vi "Graph Builder GUI - 6Dsupported.vi"() -> ()   [LabVIEW 2019]
uses:
  AxisMenu--Enum.ctl
  <vilib>/Utility/file.llb/Read Delimited Spreadsheet (string).vi
panel:
  out "Not Normalized":T1(array[cluster])
  out "Normalized":T1(array[cluster])
  out "Time Left (min)":dbl=54754.644
  out "Percent Complete":dbl(slide) scale=0.0..1.0
  in  "Axis Menu Type Def":T2 caption="Axis Menu" items=["<Ignore>", "<X Axis>", "<Y Axis>", "<Color Axis>", "<Time Axis>", "<Supra-X Scroll>", "<Supra-Y Scroll>"]
  in  "Normalize? (F)":bool
  in  "Path to Cleaned Data File":path=path "D:/Ian_s Dropbox/Dropbox/PostDoc/Programs/Data/2020-01-23 BigSlab2 Merged CLEAN  v01"
  in  "Axis Menus 2":T3={"Axis Menu 1"=1, "Axis Menu 2"=3, "Axis Menu 3"=0, "Axis Menu 4"=7, "Axis Menu 5"=9, "Axis Menu 6"=0, "Axis Menu 7"=0, "Axis Menu 8"=0, "Axis Menu 9"=4, "Axis Menu 10"=2, "Axis Menu 11"=0, "Axis Menu 12"=0} {"Axis Menu 12" items=["<Ignore>", "<X Axis>", "<Y Axis>", "<Color Axis>", "<Time Axis>", "<Supra-X Scroll>", "<Supra-Y Scroll>", "3000"]; "Axis Menu 11" items=["<Ignore>", "<X Axis>", "<Y Axis>", "<Color Axis>", "<Time Axis>", "<Supra-X Scroll>", "<Supra-Y Scroll>", "3.950000E+0", "4.300000E+0", "4.650000E+0", "5.000000E+0"]; "Axis Menu 10" items=["<Ignore>", "<X Axis>", "<Y Axis>", "<Color Axis>", "<Time Axis>", "<Supra-X Scroll>", "<Supra-Y Scroll>", "0.000000E+0"]; "Axis Menu 9" items=["<Ignore>", "<X Axis>", "<Y Axis>", "<Color Axis>", "<Time Axis>", "<Supra-X Scroll>", "<Supra-Y Scroll>", "0.000000E+0"]; "Axis Menu 8" items=["<Ignore>", "<X Axis>", "<Y Axis>", "<Color Axis>", "<Time Axis>", "<Supra-X Scroll>", "<Supra-Y Scroll>", "1.000000E-4"]; "Axis Menu 7" items=["<Ignore>", "<X Axis>", "<Y Axis>", "<Color Axis>", "<Time Axis>", "<Supra-X Scroll>", "<Supra-Y Scroll>", "1.000000E+0"]; "Axis Menu 6" items=["<Ignore>", "<X Axis>", "<Y Axis>", "<Color Axis>", "<Time Axis>", "<Supra-X Scroll>", "<Supra-Y Scroll>", "1.000000E+0", "2.000000E+0", "3.000000E+0"]; "Axis Menu 5" items=["<Ignore>", "<X Axis>", "<Y Axis>", "<Color Axis>", "<Time Axis>", "<Supra-X Scroll>", "<Supra-Y Scroll>", "9.200000E-1"]; "Axis Menu 4" items=["<Ignore>", "<X Axis>", "<Y Axis>", "<Color Axis>", "<Time Axis>", "<Supra-X Scroll>", "<Supra-Y Scroll>", "1.000000E-9", "3.500000E-1", "7.000000E-1", "1.050000E+0"]; "Axis Menu 3" items=["<Ignore>", "<X Axis>", "<Y Axis>", "<Color Axis>", "<Time Axis>", "<Supra-X Scroll>", "<Supra-Y Scroll>", "5.000000E+0"]; "Axis Menu 2" items=["<Ignore>", "<X Axis>", "<Y Axis>", "<Color Axis>", "<Time Axis>", "<Supra-X Scroll>", "<Supra-Y Scroll>", "SLAB"]; "Axis Menu 1" items=["<Ignore>", "<X Axis>", "<Y Axis>", "<Color Axis>", "<Time Axis>", "<Supra-X Scroll>", "<Supra-Y Scroll>", "2.0"]}
  in  "Color 1":u32(colorbox)
  in  "Color 2":u32(colorbox)=16711680
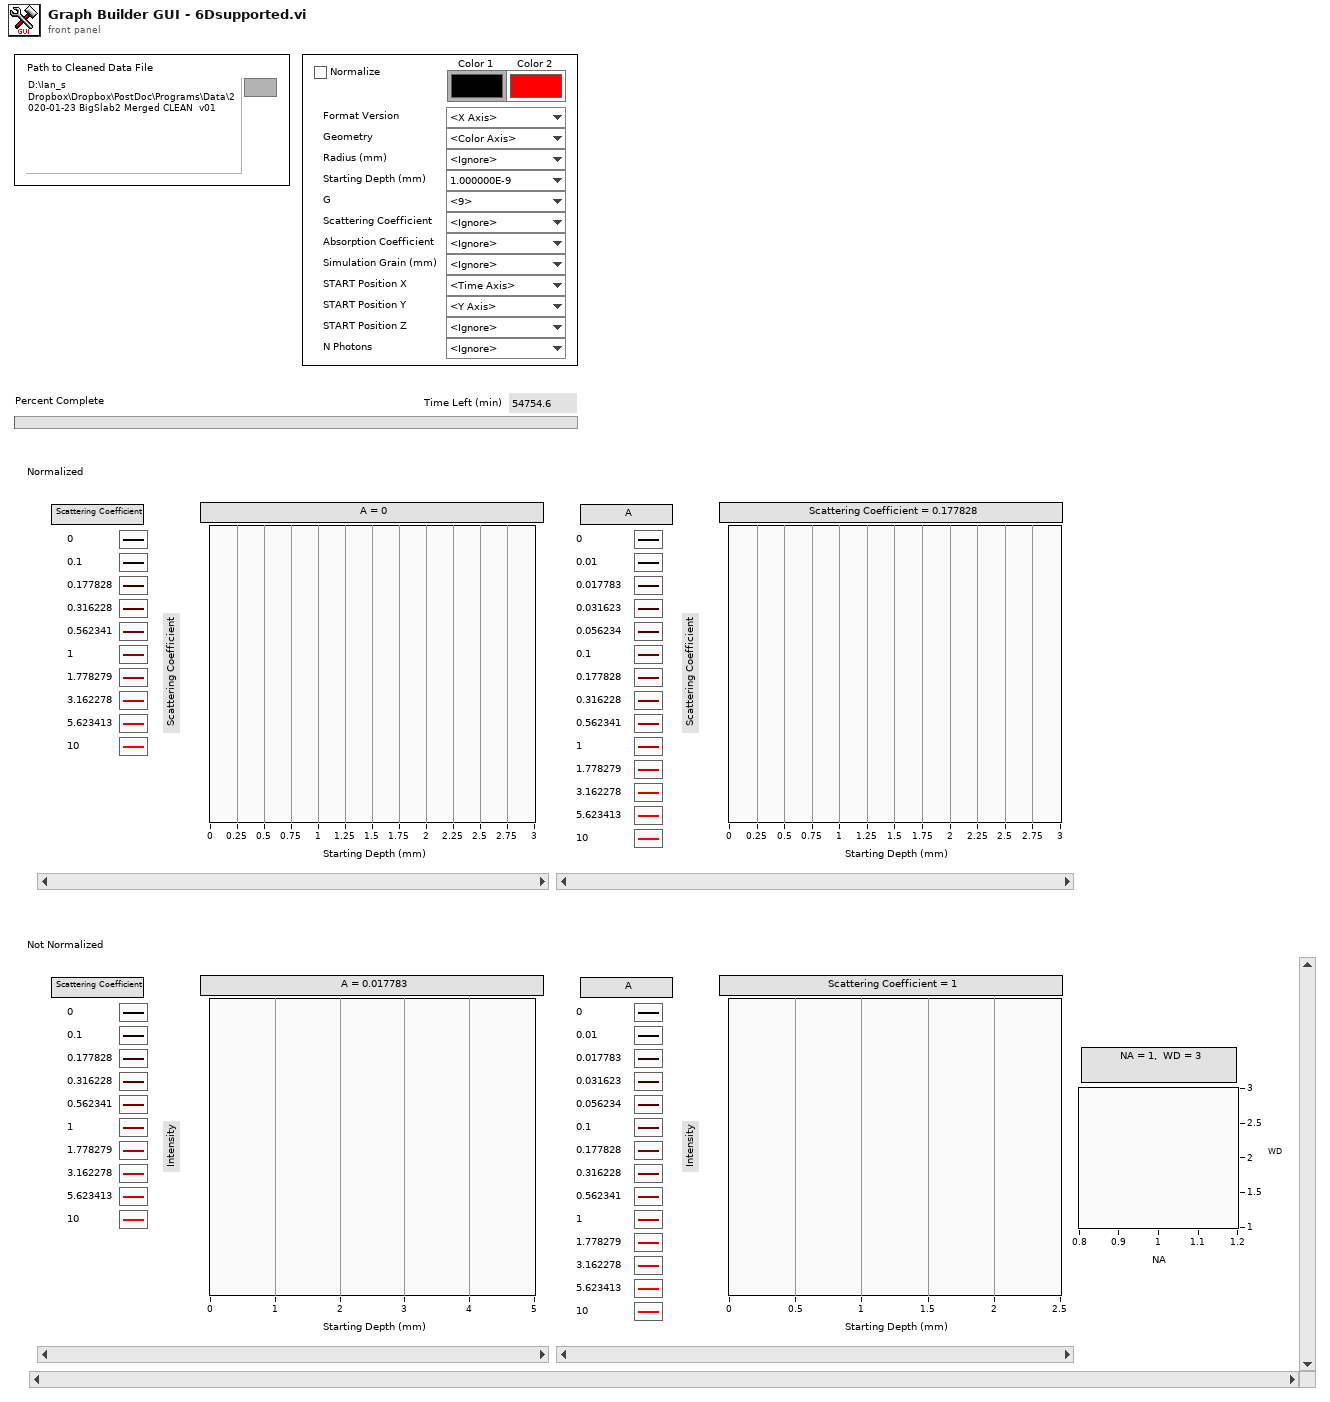
[diagram p1: front panel]
types:
  T1 = cluster{"Slab C=A, T=S 2":cluster{"Color and Time Graph":cluster{dbl[], dbl[]}[], "String":string, "String 2":string}[], "Slab C=S, T=A":cluster{"Color and Time Flipped Graph":cluster{dbl[], dbl[]}[], "String":string, "String 2":string}[], "Supra-Space Label":string, "Supra-Space Mini Map":cluster{dbl[], dbl[]}[]}[][]
  T2 = typedef "AxisMenu--Enum.ctl" = u16
  T3 = cluster{"Axis Menu 1":u16, "Axis Menu 2":u16, "Axis Menu 3":u16, "Axis Menu 4":u16, "Axis Menu 5":u16, "Axis Menu 6":u16, "Axis Menu 7":u16, "Axis Menu 8":u16, "Axis Menu 9":u16, "Axis Menu 10":u16, "Axis Menu 11":u16, "Axis Menu 12":u16}
  T4 = cluster{cluster{dbl[], dbl[]}[], string, "Caption.Text":string}[]
  T5 = cluster{"Graph":cluster{cluster{dbl[], dbl[]}[], string, "Caption.Text":string}[], "Graph":cluster{cluster{dbl[], dbl[]}[], string, "Caption.Text":string}[], string, cluster{dbl[], dbl[]}[]}
  T6 = cluster{"Graph":cluster{cluster{dbl[], dbl[]}[], string, "Caption.Text":string}[], "Graph":cluster{cluster{dbl[], dbl[]}[], string, "Caption.Text":string}[], string, cluster{dbl[], dbl[]}[]}[][]
  T7 = cluster{"Graph":cluster{cluster{dbl[], dbl[]}[], string, "Caption.Text":string}[], "Graph":cluster{cluster{dbl[], dbl[]}[], string, "Caption.Text":string}[], string, "XY Graph in Array":cluster{i32[], i32[]}[]}
  T8 = cluster{"Graph":cluster{cluster{dbl[], dbl[]}[], string, "Caption.Text":string}[], "Graph":cluster{cluster{dbl[], dbl[]}[], string, "Caption.Text":string}[], string, "XY Graph in Array":cluster{i32[], i32[]}[]}[]
  T9 = cluster{"Graph":cluster{cluster{dbl[], dbl[]}[], string, "Caption.Text":string}[], "Graph":cluster{cluster{dbl[], dbl[]}[], string, "Caption.Text":string}[], string, "XY Graph in Array":cluster{i32[], i32[]}[]}[][]
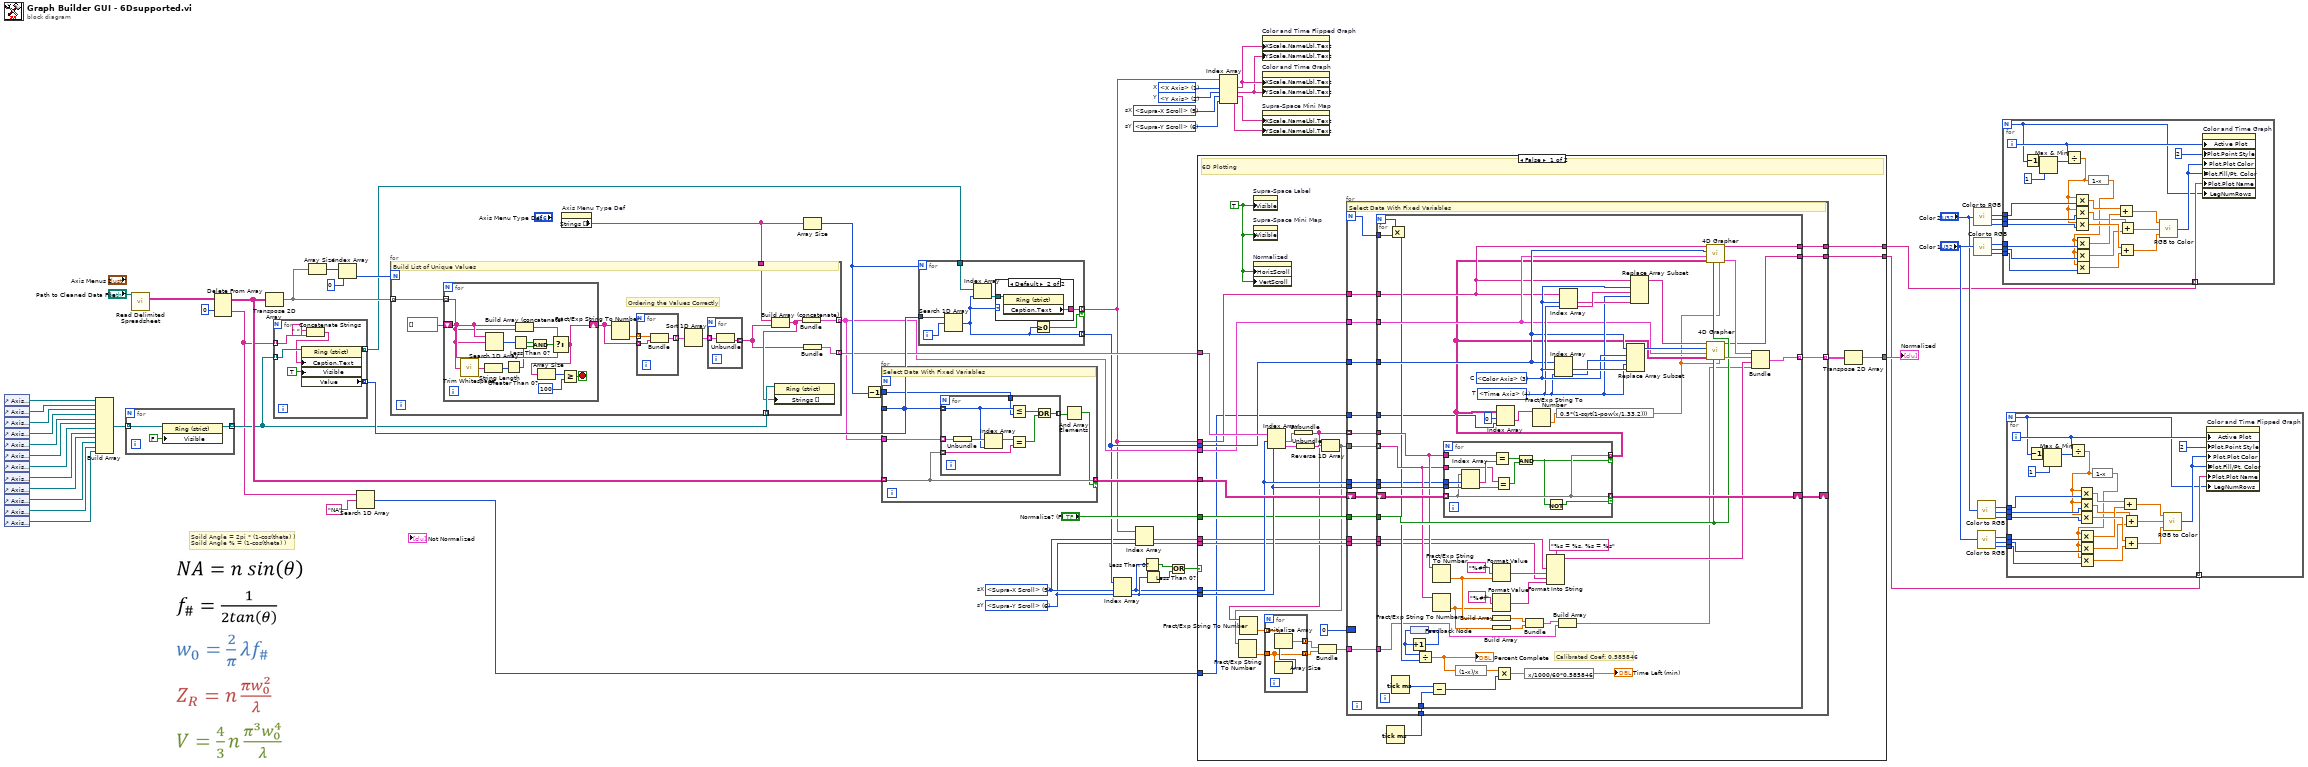
[diagram p0: block diagram]
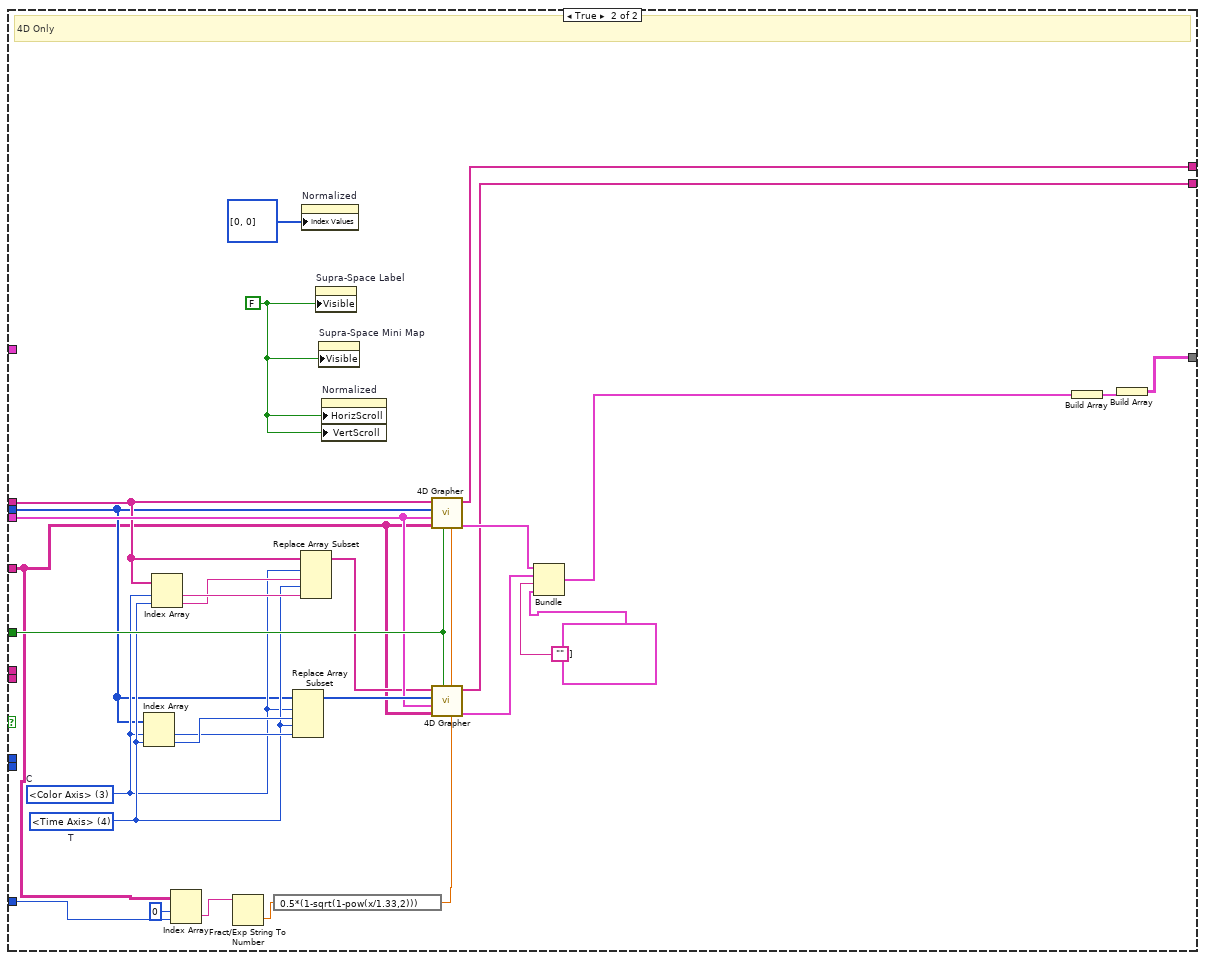
[diagram p2: hidden frame]
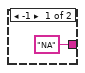
[diagram p3: hidden frame]
diagram:
  w6 = T2 1 items=["<Ignore>", "<X Axis>", "<Y Axis>", "<Color Axis>", "<Time Axis>", "<Supra-X Scroll>", "<Supra-Y Scroll>"]  # X
  w9 = T2 6 items=["<Ignore>", "<X Axis>", "<Y Axis>", "<Color Axis>", "<Time Axis>", "<Supra-X Scroll>", "<Supra-Y Scroll>"]  # sY
  w10 = T2 5 items=["<Ignore>", "<X Axis>", "<Y Axis>", "<Color Axis>", "<Time Axis>", "<Supra-X Scroll>", "<Supra-Y Scroll>"]  # sX
  w13 = T2 6 items=["<Ignore>", "<X Axis>", "<Y Axis>", "<Color Axis>", "<Time Axis>", "<Supra-X Scroll>", "<Supra-Y Scroll>"]  # sY
  w14 = T2 5 items=["<Ignore>", "<X Axis>", "<Y Axis>", "<Color Axis>", "<Time Axis>", "<Supra-X Scroll>", "<Supra-Y Scroll>"]  # sX
  w46 = T2 2 items=["<Ignore>", "<X Axis>", "<Y Axis>", "<Color Axis>", "<Time Axis>", "<Supra-X Scroll>", "<Supra-Y Scroll>"]  # Y
  # "Soild Angle = 2pi * (1-cos(theta) )\nSoild Angle % = (1-cos(theta) )"
  n1 = control-ref of="Axis Menu 1"() -> (w51:refnum<vi>)
  n2 = control-ref of="Axis Menu 2"() -> (w66:refnum<vi>)
  n3 = control-ref of="Axis Menu 3"() -> (w65:refnum<vi>)
  n4 = control-ref of="Axis Menu 4"() -> (w64:refnum<vi>)
  n5 = control-ref of="Axis Menu 5"() -> (w63:refnum<vi>)
  n6 = control-ref of="Axis Menu 6"() -> (w62:refnum<vi>)
  n7 = control-ref of="Axis Menu 7"() -> (w61:refnum<vi>)
  n8 = control-ref of="Axis Menu 8"() -> (w60:refnum<vi>)
  n9 = control-ref of="Axis Menu 9"() -> (w59:refnum<vi>)
  n10 = control-ref of="Axis Menu 10"() -> (w58:refnum<vi>)
  n11 = control-ref of="Axis Menu 11"() -> (w57:refnum<vi>)
  n12 = control-ref of="Axis Menu 12"() -> (w56:refnum<vi>)
  n13 = Build Array(w51, w66, w65, w64, w63, w62, w61, w60, w59, w58, w57, w56) -> (w55:refnum<vi>[])
  n14 = for {
    tunnel: w55 -> [w73] mode=indexing
    tunnel: [w71] -> w44 mode=indexing
    n15 = property on="Property Node" class="Ring (strict)"(reference=w73, "Visible"=FALSE) -> (reference out=w71:refnum<vi>)  [unwired: 1 in, 1 out]
  }
  n16 = call-poly <vilib>:"Read Delimited Spreadsheet.vi"("file path (dialog if empty)"="Path to Cleaned Data File") -> ("all rows"=w52:string[][])  [unwired: 9 in, 5 out]
  n17 = Delete From Array(array=w52, index (row)=0) -> (deleted portion=w3:string[], array with subset deleted=w50:string[][])  [unwired: 2 in]
  n18 = Transpose 2D Array(2D array=w50) -> (transposed array=w68:string[][])
  n19 = for {
    tunnel: w3 -> [w76] mode=indexing
    tunnel: w44 -> [w80] mode=indexing
    tunnel: [w78] -> w47 mode=indexing
    tunnel: [w77] -> w45 mode=indexing
    n20 = Concatenate Strings(" " ("string"), w76) -> (w74:string)
    n21 = property on="Property Node" class="Ring (strict)"(reference=w80, "Caption.Text"=w74, "Visible"=TRUE) -> (reference out=w77:refnum<vi>, "Value"=w78:u16)  [unwired: 1 in, 1 out]
  }
  n22 = Array Size(array=w68) -> (size(s)=w69:i32[])
  n23 = Index Array(array=w69, index=0) -> (element=w54:i32)
  n24 = Search 1D Array(1D array=w3, element="NA") -> (index of element=w1:i32)  [unwired: 1 in]
  n25 = property on="Axis Menu Type Def" class="Ring (strict)"() -> ("Strings []"=w49:string[])  [unwired: 2 in, 2 out]
  n26 = for {
    N: w54 -> [_]
    tunnel: w68 -> [w92] mode=indexing
    tunnel: [w90] -> w34 mode=indexing
    tunnel: w49 -> [w89]
    tunnel: w44 -> [w88] mode=indexing
    tunnel: [w86] -> w37 mode=indexing
    # "Ordering the Values Correctly"
    # "Build List of Unique Values"
    n27 = for {
      tunnel: w92 -> [w99] mode=indexing
      shift-right: [w106] -> w82
      shift-left: string[] [] -> [w110]
      stop <- w103 stop-if-true
      n28 = call <vilib>:"Trim Whitespace.vi"("string"=w99) -> ("trimmed string"=w98:string)  [unwired: 1 in]
      n29 = String Length(string=w98) -> (length=w102:i32)
      n30 = Search 1D Array(1D array=w110, element=w99) -> (index of element=w108:i32)  [unwired: 1 in]
      n31 = Greater Than 0?(x=w102) -> (x > 0?=w100:bool)
      n32 = Less Than 0?(x=w108) -> (x < 0?=w107:bool)
      n33 = Build Array (concatenate)(w110, w99) -> (w109:string[])
      n34 = And(x=w107, y=w100) -> (x .and. y?=w101:bool)
      n35 = Select(t=w109, s=w101, f=w110) -> (s? t:f=w106:string[])
      n36 = Array Size(array=w106) -> (size(s)=w105:i32)
      n37 = Greater Or Equal?(x=w105, y=100) -> (x >= y?=w103:bool)
    }
    n38 = Fract/Exp String To Number(string=w82) -> (number=w85:dbl[])  [unwired: 3 in, 1 out]
    n39 = for {
      tunnel: w85 -> [w97] mode=indexing
      tunnel: w82 -> [w96] mode=indexing
      tunnel: [w95] -> w84 mode=indexing
      n40 = Bundle(w97, w96) -> (w95:cluster{dbl, string})  [unwired: 1 in]
    }
    n41 = Sort 1D Array(array=w84) -> (sorted array=w83:cluster{dbl, string}[])
    n42 = for {
      tunnel: w83 -> [w94] mode=indexing
      tunnel: [w93] -> w81 mode=indexing
      n43 = Unbundle(w94) -> (w93:string)  [unwired: 1 out]
    }
    n44 = Build Array (concatenate)(w89, w81) -> (w87:string[])
    n45 = property on="Property Node" class="Ring (strict)"(reference=w88, "Strings []"=w87) -> ()  [unwired: 1 in, 2 out]
    n46 = Bundle(w87) -> (w90:cluster{string[]})  [unwired: 1 in]
    n47 = Bundle(w81) -> (w86:cluster{string[]})  [unwired: 1 in]
  }
  n48 = Array Size(array=w49) -> (size(s)=w43:i32)
  n49 = Decrement(x=w43) -> (x-1=w48:i32)
  n50 = for {
    tunnel: w50 -> [w115] mode=indexing
    tunnel: [w115] -> w35 mode=indexing if=w112
    tunnel: w47 -> [w116]
    tunnel: w34 -> [w114]
    tunnel: w48 -> [w111]
    # "Select Data With Fixed Variables"
    n51 = for {
      tunnel: w116 -> [w121] mode=indexing
      tunnel: w115 -> [w123] mode=indexing
      tunnel: w114 -> [w125] mode=indexing
      tunnel: [w118] -> w113 mode=indexing
      tunnel: w111 -> [w117]
      n52 = Unbundle(w125) -> (w124:string[])
      n53 = Index Array(array=w124, index=w121) -> (element=w122:string)
      n54 = Less Or Equal?(x=w121, y=w117) -> (x <= y?=w120:bool)
      n55 = Equal?(x=w122, y=w123) -> (x = y?=w119:bool)
      n56 = Or(x=w120, y=w119) -> (x .or. y?=w118:bool)
    }
    n57 = And Array Elements(Boolean array=w113) -> (logical AND=w112:bool)
  }
  n58 = for {
    N: w43 -> [_]
    tunnel: w47 -> [w132]
    tunnel: [w127] -> w33 mode=indexing
    tunnel: w45 -> [w129]
    tunnel: [w128] -> w15 mode=indexing if=w126
    i -> [w131]
    n59 = Search 1D Array(1D array=w132, element=w131) -> (index of element=w127:i32)  [unwired: 1 in]
    n60 = Index Array(array=w129, index=w127) -> (element=w130:refnum<vi>)
    n61 = case shown="Default" w127 {
      tunnel: w130 -> [_ w135]
      tunnel: ["NA" ("Caption.Text") w134] -> w128
      frame -1 {
      }
      frame Default {
        n62 = property on="Property Node" class="Ring (strict)"(reference=w135) -> ("Caption.Text"=w134:string)  [unwired: 1 in, 2 out]
      }
    }
    n63 = Greater Or Equal To 0?(x=w127) -> (x >= 0?=w126:bool)
  }
  n64 = Index Array(array=w33, index #1=w14, index #2=w13) -> (element #1=w38:i32, element #2=w39:i32)
  n65 = Index Array(array=w15, index #1=w14, index #2=w13) -> (element #1=w12:string, element #2=w11:string)
  n66 = Less Than 0?(x=w38) -> (x < 0?=w41:bool)
  n67 = Less Than 0?(x=w39) -> (x < 0?=w42:bool)
  n68 = Or(x=w41, y=w42) -> (x .or. y?=w40:bool)
  n69 = case shown="False" w40 {
    tunnel: "Normalize? (F)" -> [w154 w279]
    tunnel: w34 -> [w156 w278]
    tunnel: w35 -> [w163 w259]
    tunnel: w15 -> [w155 w273]
    tunnel: w33 -> [w157 w271]
    tunnel: w39 -> [w158 _]
    tunnel: w38 -> [w162 _]
    tunnel: w37 -> [w160 _]
    tunnel: [w142 w269] -> w32
    tunnel: [w151 w264] -> w17
    tunnel: [w150 w263] -> w16
    tunnel: w12 -> [w141 _]
    tunnel: w11 -> [w140 _]
    tunnel: w1 -> [w136 w258]
    frame False {
      w137 = TRUE ("Visible")
      # "6D Plotting"
      n70 = property on="Supra-Space Label" class="Str"("Visible"=w137) -> ()  [unwired: 2 in, 2 out]
      n71 = property on="Supra-Space Mini Map" class="XYGraph (strict)"("Visible"=w137) -> ()  [unwired: 2 in, 2 out]
      n72 = property on="Normalized" class="Arr (strict)"("HorizScroll"=w137, "VertScroll"=w137) -> ()  [unwired: 2 in, 2 out]
      n73 = Index Array(array=w160, index #1=w162, index #2=w158) -> (element #1=w161:cluster{string[]}, element #2=w159:cluster{string[]})
      n74 = Unbundle(w161) -> (w139:string[])
      n75 = Fract/Exp String To Number(string=w139) -> (number=w148:dbl[])  [unwired: 3 in, 1 out]
      n76 = Unbundle(w159) -> (w149:string[])
      n77 = Reverse 1D Array(array=w149) -> (reversed array=w138:string[])
      n78 = Fract/Exp String To Number(string=w138) -> (number=w147:dbl[])  [unwired: 3 in, 1 out]
      n79 = for {
        tunnel: w148 -> [w167] mode=indexing
        tunnel: w147 -> [w164]
        tunnel: [w166] -> w145 mode=concatenating
        tunnel: [w164] -> w144 mode=concatenating
        n80 = Array Size(array=w164) -> (size(s)=w165:i32)
        n81 = Initialize Array(w167, w165) -> (w166:dbl[])
      }
      n82 = Bundle(w145, w144) -> (w143:cluster{dbl[], dbl[]})  [unwired: 1 in]
      n83 = Tick Count (ms)() -> (millisecond timer value=w153:u32)
      n84 = for {
        N -> [w172]
        tunnel: w162 -> [w185]
        tunnel: w138 -> [w183]
        tunnel: w139 -> [w184] mode=indexing
        shift-right: [w181] -> _
        shift-left: w163 -> [w186]
        tunnel: w158 -> [w182]
        tunnel: w156 -> [w180]
        tunnel: w155 -> [w179]
        tunnel: w157 -> [w178]
        tunnel: w154 -> [w177]
        tunnel: w153 -> [w176]
        tunnel: [w175] -> w152 mode=indexing
        tunnel: [w174] -> w151
        tunnel: [w173] -> w150
        border: 0 -> [_]
        tunnel: w143 -> [w171]
        tunnel: w141 -> [w170]
        tunnel: w140 -> [w169]
        tunnel: w136 -> [w168]
        # "Select Data With Fixed Variables"
        n85 = for {
          N -> [w226]
          tunnel: w185 -> [w195]
          tunnel: w184 -> [w215]
          tunnel: w183 -> [w213] mode=indexing
          shift-right: [w240] -> w181
          shift-left: w186 -> [w242]
          tunnel: w182 -> [w241]
          tunnel: w180 -> [w227]
          tunnel: w179 -> [w196]
          tunnel: w178 -> [w229]
          tunnel: w177 -> [w228]
          tunnel: w176 -> [w224]
          tunnel: [w211] -> w175 mode=indexing
          tunnel: [w209] -> w174
          tunnel: [w208] -> w173
          tunnel: w172 -> [w206]
          tunnel: w171 -> [w199]
          tunnel: w170 -> [w194]
          tunnel: w169 -> [w193]
          tunnel: w168 -> [w188]
          w230 = T2 4 items=["<Ignore>", "<X Axis>", "<Y Axis>", "<Color Axis>", "<Time Axis>", "<Supra-X Scroll>", "<Supra-Y Scroll>"]  # T
          w231 = T2 3 items=["<Ignore>", "<X Axis>", "<Y Axis>", "<Color Axis>", "<Time Axis>", "<Supra-X Scroll>", "<Supra-Y Scroll>"]  # C
          # "Calibrated Coef: 0.585846"
          n86 = Multiply(x=w226, y=w206) -> (x*y=w207:i32)
          n87 = Tick Count (ms)() -> (millisecond timer value=w225:u32)
          n88 = feedback #1() -> (w204:i32)
          n89 = Increment(x=w204) -> (x+1=w205:i32)
          n90 = feedback-in #1(w205) -> ()
          n91 = Divide(x=w204, y=w207) -> (x/y=w223:dbl)
          "Percent Complete" <- w223
          n92 = Subtract(x=w225, y=w224) -> (x-y=w221:u32)
          n93 = Fract/Exp String To Number(string=w215) -> (number=w203:dbl)  [unwired: 3 in, 1 out]
          n94 = Fract/Exp String To Number(string=w213) -> (number=w202:dbl)  [unwired: 3 in, 1 out]
          n95 = for {
            tunnel: w242 -> [w245] mode=indexing
            tunnel: w215 -> [w253]
            tunnel: w213 -> [w248]
            tunnel: w241 -> [w252]
            tunnel: w195 -> [w251]
            tunnel: [w245] -> w240 mode=indexing if=w243
            tunnel: [w245] -> w189 mode=indexing if=w244
            n96 = Index Array(array=w245, index #1=w251, index #2=w252) -> (element #1=w249:string, element #2=w250:string)
            n97 = Equal?(x=w253, y=w249) -> (x = y?=w246:bool)
            n98 = Equal?(x=w248, y=w250) -> (x = y?=w247:bool)
            n99 = And(x=w246, y=w247) -> (x .and. y?=w244:bool)
            n100 = Not(x=w244) -> (.not. x?=w243:bool)
          }
          n101 = expression code="(1-x)/x"(w223) -> (w222:dbl)
          n102 = Format Value(format string="%#f", value (0)=w203) -> (output string=w218:string)  [unwired: 1 in]
          n103 = Build Array(w203) -> (w201:dbl[])
          n104 = Build Array(w202) -> (w200:dbl[])
          n105 = Format Value(format string="%#f", value (0)=w202) -> (output string=w212:string)  [unwired: 1 in]
          n106 = Multiply(x=w222, y=w221) -> (x*y=w220:dbl)
          n107 = Index Array(array=w189, index (row)=0 ("disabled index (row)"), index (col)=w188) -> (element=w191:string)
          n108 = expression code="x/1000/60*0.585846"(w220) -> (→"Time Left (min)":dbl)
          n109 = Bundle(w201, w200) -> (w198:cluster{dbl[], dbl[]})  [unwired: 1 in]
          n110 = Fract/Exp String To Number(string=w191) -> (number=w190:dbl)  [unwired: 3 in, 1 out]
          n111 = Format Into String(format string="%s = %s, %s = %s", w194, w218, w193, w212) -> (resulting string=w210:string)  [unwired: 2 in, 1 out]
          n112 = Index Array(array=w229, index #1=w231, index #2=w230) -> (element #1=w233:i32, element #2=w232:i32)
          n113 = expression code="0.5*(1-sqrt(1-pow(x/1.33,2)))"(w190) -> (w187:dbl)
          n114 = Build Array(w198, w199) -> (w197:cluster{dbl[], dbl[]}[])
          n115 = Index Array(array=w196, index #1=w231, index #2=w230) -> (element #1=w234:string, element #2=w235:string)
          n116 = Replace Array Subset(array=w229, new element #1=w232, index #1=w231, new element #2=w233, index #2=w230) -> (w237:i32[])
          n117 = Replace Array Subset(array=w196, new element #1=w235, index #1=w231, new element #2=w234, index #2=w230) -> (w236:string[])
          n118 = call "4D Grapher.vi"("Norm Factor (NaN: use first element)"=w187, "Normalize? (F)"=w228, "Pruned Data"=w189, "String Items from Axes Menus"=w227, "Axes Indexes"=w229, "Axes Names"=w196) -> ("Graph"=w239:T4, "Color Axis Titles"=w209:string[])  [unwired: 4 in]
          n119 = call "4D Grapher.vi"("Norm Factor (NaN: use first element)"=w187, "Normalize? (F)"=w228, "Pruned Data"=w189, "String Items from Axes Menus"=w227, "Axes Indexes"=w237, "Axes Names"=w236) -> ("Graph"=w238:T4, "Color Axis Titles"=w208:string[])  [unwired: 4 in]
          n120 = Bundle("Graph"=w239, "Graph"=w238, w210, w197) -> (w211:T5)  [unwired: 1 in]
        }
      }
      n121 = Transpose 2D Array(2D array=w152) -> (transposed array=w142:T6)
    }
    frame True {
      w260 = FALSE ("Visible")
      w275 = T2 4 items=["<Ignore>", "<X Axis>", "<Y Axis>", "<Color Axis>", "<Time Axis>", "<Supra-X Scroll>", "<Supra-Y Scroll>"]  # T
      w274 = T2 3 items=["<Ignore>", "<X Axis>", "<Y Axis>", "<Color Axis>", "<Time Axis>", "<Supra-X Scroll>", "<Supra-Y Scroll>"]  # C
      # "4D Only"
      n122 = Index Array(array=w271, index #1=w274, index #2=w275) -> (element #1=w281:i32, element #2=w282:i32)
      n123 = Index Array(array=w273, index #1=w274, index #2=w275) -> (element #1=w277:string, element #2=w276:string)
      n124 = Index Array(array=w259, index (row)=0 ("disabled index (row)"), index (col)=w258) -> (element=w256:string)
      n125 = Fract/Exp String To Number(string=w256) -> (number=w255:dbl)  [unwired: 3 in, 1 out]
      n126 = expression code="0.5*(1-sqrt(1-pow(x/1.33,2)))"(w255) -> (w254:dbl)
      n127 = Replace Array Subset(array=w271, new element #1=w282, index #1=w274, new element #2=w281, index #2=w275) -> (w280:i32[])
      n128 = Replace Array Subset(array=w273, new element #1=w276, index #1=w274, new element #2=w277, index #2=w275) -> (w272:string[])
      n129 = property on="Normalized" class="Arr (strict)"("Index Values"=u32[] [0, 0]) -> ()  [unwired: 2 in, 2 out]
      n130 = property on="Supra-Space Label" class="Str"("Visible"=w260) -> ()  [unwired: 2 in, 2 out]
      n131 = property on="Supra-Space Mini Map" class="XYGraph (strict)"("Visible"=w260) -> ()  [unwired: 2 in, 2 out]
      n132 = property on="Normalized" class="Arr (strict)"("HorizScroll"=w260, "VertScroll"=w260) -> ()  [unwired: 2 in, 2 out]
      n133 = call "4D Grapher.vi"("Norm Factor (NaN: use first element)"=w254, "Normalize? (F)"=w279, "Pruned Data"=w259, "String Items from Axes Menus"=w278, "Axes Indexes"=w271, "Axes Names"=w273) -> ("Graph"=w268:T4, "Color Axis Titles"=w264:string[])  [unwired: 4 in]
      n134 = call "4D Grapher.vi"("Norm Factor (NaN: use first element)"=w254, "Normalize? (F)"=w279, "Pruned Data"=w259, "String Items from Axes Menus"=w278, "Axes Indexes"=w280, "Axes Names"=w272) -> ("Graph"=w267:T4, "Color Axis Titles"=w263:string[])  [unwired: 4 in]
      n135 = Bundle("Graph"=w268, "Graph"=w267, "", "XY Graph in Array"=cluster{i32[], i32[]}[] []) -> (w265:T7)  [unwired: 1 in]
      n136 = Build Array(w265) -> (w270:T8)
      n137 = Build Array(w270) -> (w269:T9)
    }
  }
  "Normalized" <- w32
  n138 = Index Array(array=w15, index #1=w6, index #2=w46, index #3=w10, index #4=w9) -> (element #1=w5:string, element #2=w4:string, element #3=w8:string, element #4=w7:string)
  n139 = property on="Color and Time Flipped Graph" class="XYGraph (strict)"("XScale.NameLbl.Text"=w5, "YScale.NameLbl.Text"=w4) -> ()  [unwired: 2 in, 2 out]
  n140 = property on="Color and Time Graph" class="XYGraph (strict)"("XScale.NameLbl.Text"=w5, "YScale.NameLbl.Text"=w4) -> ()  [unwired: 2 in, 2 out]
  n141 = property on="Supra-Space Mini Map" class="XYGraph (strict)"("XScale.NameLbl.Text"=w8, "YScale.NameLbl.Text"=w7) -> ()  [unwired: 2 in, 2 out]
  n142 = call <vilib>:"Color to RGB.vi"("Color"="Color 2") -> ("R"=w18:u8, "G"=w19:u8, "B"=w20:u8)  [unwired: 1 out]
  n143 = call <vilib>:"Color to RGB.vi"("Color"="Color 1") -> ("R"=w21:u8, "G"=w22:u8, "B"=w23:u8)  [unwired: 1 out]
  n144 = call <vilib>:"Color to RGB.vi"("Color"="Color 2") -> ("R"=w29:u8, "G"=w28:u8, "B"=w27:u8)  [unwired: 1 out]
  n145 = call <vilib>:"Color to RGB.vi"("Color"="Color 1") -> ("R"=w26:u8, "G"=w25:u8, "B"=w24:u8)  [unwired: 1 out]
  n146 = for {
    N -> [w285]
    tunnel: w18 -> [w304]
    tunnel: w19 -> [w303]
    tunnel: w20 -> [w302]
    tunnel: w21 -> [w301]
    tunnel: w22 -> [w300]
    tunnel: w23 -> [w299]
    tunnel: w17 -> [w286] mode=indexing
    i -> [w306]
    n147 = Decrement(x=w285) -> (x-1=w305:i32)
    n148 = Max & Min(x=w305, y=1) -> (max(x,y)=w284:i32)  [unwired: 1 out]
    n149 = Divide(x=w306, y=w284) -> (x/y=w298:dbl)
    n150 = Multiply(x=w298, y=w304) -> (x*y=w292:dbl)
    n151 = Multiply(x=w298, y=w303) -> (x*y=w293:dbl)
    n152 = Multiply(x=w298, y=w302) -> (x*y=w296:dbl)
    n153 = expression code="1-x"(w298) -> (w288:dbl)
    n154 = Multiply(x=w288, y=w301) -> (x*y=w294:dbl)
    n155 = Multiply(x=w288, y=w300) -> (x*y=w295:dbl)
    n156 = Multiply(x=w288, y=w299) -> (x*y=w297:dbl)
    n157 = Add(x=w292, y=w294) -> (x+y=w291:dbl)
    n158 = Add(x=w296, y=w297) -> (x+y=w289:dbl)
    n159 = Add(x=w293, y=w295) -> (x+y=w290:dbl)
    n160 = call <vilib>:"RGB to Color.vi"("B"=w289, "G"=w290, "R"=w291) -> ("Color"=w287:u32)
    n161 = property on="Color and Time Graph" class="XYGraph (strict)"("Active Plot"=w306, "Plot.Point Style"=u8 2, "Plot.Plot Color"=w287, "Plot.Fill/Pt. Color"=w287, "Plot.Plot Name"=w286, "LegNumRows"=w285) -> ()  [unwired: 2 in, 2 out]
  }
  n162 = for {
    N -> [w310]
    tunnel: w29 -> [w329]
    tunnel: w28 -> [w328]
    tunnel: w27 -> [w327]
    tunnel: w26 -> [w326]
    tunnel: w25 -> [w325]
    tunnel: w24 -> [w324]
    tunnel: w16 -> [w311] mode=indexing
    i -> [w331]
    n163 = Decrement(x=w310) -> (x-1=w330:i32)
    n164 = Max & Min(x=w330, y=1) -> (max(x,y)=w309:i32)  [unwired: 1 out]
    n165 = Divide(x=w331, y=w309) -> (x/y=w323:dbl)
    n166 = Multiply(x=w323, y=w329) -> (x*y=w317:dbl)
    n167 = Multiply(x=w323, y=w328) -> (x*y=w318:dbl)
    n168 = Multiply(x=w323, y=w327) -> (x*y=w321:dbl)
    n169 = expression code="1-x"(w323) -> (w313:dbl)
    n170 = Multiply(x=w313, y=w326) -> (x*y=w319:dbl)
    n171 = Multiply(x=w313, y=w325) -> (x*y=w320:dbl)
    n172 = Multiply(x=w313, y=w324) -> (x*y=w322:dbl)
    n173 = Add(x=w317, y=w319) -> (x+y=w316:dbl)
    n174 = Add(x=w321, y=w322) -> (x+y=w314:dbl)
    n175 = Add(x=w318, y=w320) -> (x+y=w315:dbl)
    n176 = call <vilib>:"RGB to Color.vi"("B"=w314, "G"=w315, "R"=w316) -> ("Color"=w312:u32)
    n177 = property on="Color and Time Flipped Graph" class="XYGraph (strict)"("Active Plot"=w331, "Plot.Point Style"=u8 2, "Plot.Plot Color"=w312, "Plot.Fill/Pt. Color"=w312, "Plot.Plot Name"=w311, "LegNumRows"=w310) -> ()  [unwired: 2 in, 2 out]
  }
